vi "Alyssa_GlueLineAndDots.vi"() -> ()   [LabVIEW 2016]
uses:
  C:/Users/Aerotech/Documents/BNLStaveAssembly-blueprint/Bin/Aerotech.A3200.dll
  BNLStaveAssembly-blueprint/Bin/Aerotech.A3200.dll
  <vilib>/vision/Image Controls.llb/IMAQ Image.ctl
  <vilib>/LabVIEW Interface for Arduino/Type Defs/Arduino Resource.ctl
  <vilib>/LabVIEW Interface for Arduino/Type Defs/Board Type.ctl
  <vilib>/LabVIEW Interface for Arduino/Type Defs/Pin Mode.ctl
  <vilib>/Utility/file.llb/Read Delimited Spreadsheet (DBL).vi
  <vilib>/LabVIEW Interface for Arduino/LabVIEW Interface for Arduino.lvlib
panel:
  out "check":dbl[][](array[numeric])
  in  "y dist (mm)":dbl
  in  "How many lines? (actual # will be x2)":i32
  in  "?":T1(tab)
  in  "Module corner coordinates":T2={"X [mm]"=-325.4922095457569, "Y [mm]"=111.42987050829626, "Z [mm] "=34.99996599632762}
  in  "Axis speeds (mm/s)":T3={"vX [mm]"=49.0, "vY [mm]"=49.0, "vZ [mm] "=49.0}
  in  "Home?":bool
  in  "Lowest Z Position":dbl=38.0
  out "Arduino Resource":T4={"VISA resource"="GlueCTRL", "Board Type"=enum."Uno", "Connection Type"=enum."USB / Serial", "Bytes Per Packet (15)"=15}
  in  "Digital I/O Pin":u8=7
  in  "XYZ Stage Control":refnum<k24>
  in  "Testing?":bool
  out "Difference camera/syringe in X":dbl=-133.03368290747076
  out "Difference camera/syringe in y":dbl=-2.170984960815403
  in  "um/pix resolution":dbl=1.58
  in  "Image Feed":T6=refnum
  in  "Path to save collected images":path=path "C:/Users/Aerotech/cernbox/BNL/Stave Assembly Records/2017-06-12/3"
  in  "Estimate distance y":dbl
  in  "Estimate distance x":dbl=130.0
  in  "Lowest Z position Calibration":dbl=17.0
  out "Final Position":T7={"Final X"=-325.49379764644783, "Final Y"=23.533617154160947, "Final Z"=34.99956596392527}
  in  "error in":errorcluster
  out "Arduino Resource 2":T4={"VISA resource"="COM4", "Board Type"=enum."Uno", "Connection Type"=enum."USB / Serial", "Bytes Per Packet (15)"=15}
  out "Module Start":T7
  in  "Digital I/O Pin 2":u8=7
  out "XYZ .NET Refnum out":refnum<k24>
  out "XYZ .NET Refnum out 2":refnum<k24>
  out "error out":errorcluster={"status"=FALSE, "code"=1073676418, "source"="VISA Close in GlueSingleModule(SubVI).vi->2_VisualizeModulePositioning2.vi->VMP_TestStand.vi"}
  # "Overview: This takes a pattern of zeroes/ones (.csv file) as well as the start coordinates of the top left corner of a module and places dots of glue  \nRequirements: NI Arduino dependencies\nInstructions: Select a .csv file (ones indicate regions for glue) as well as a starting coordinate (this is default to the top left corner of the module spacer). You \ncan also input axis speeds (default to maximum) and module lengths and widths (default to 90 mm) which are the widths of the module to which you want to \nplace glue. Lastly, one can choose to Home the stage here and can select the lowest position in Z. The default is that the stage moves down 2-3 mm in Z \nwhile dispensing.  The Arduino inputs are default and simply allow the LabView program to drigger the Arduino (which sends a signal to the dispenser). The \nprogram signals to dispense air- all other parameters such as length of dispensing (default: 350 millisec), pressure (default: 48 psi), and vacuum pressure \n(default: 7.8 psi) are set on the dispenser itself. The defaults are highly recommended here."
  # "Positioning Inputs"
  # "Arduino Inputs"
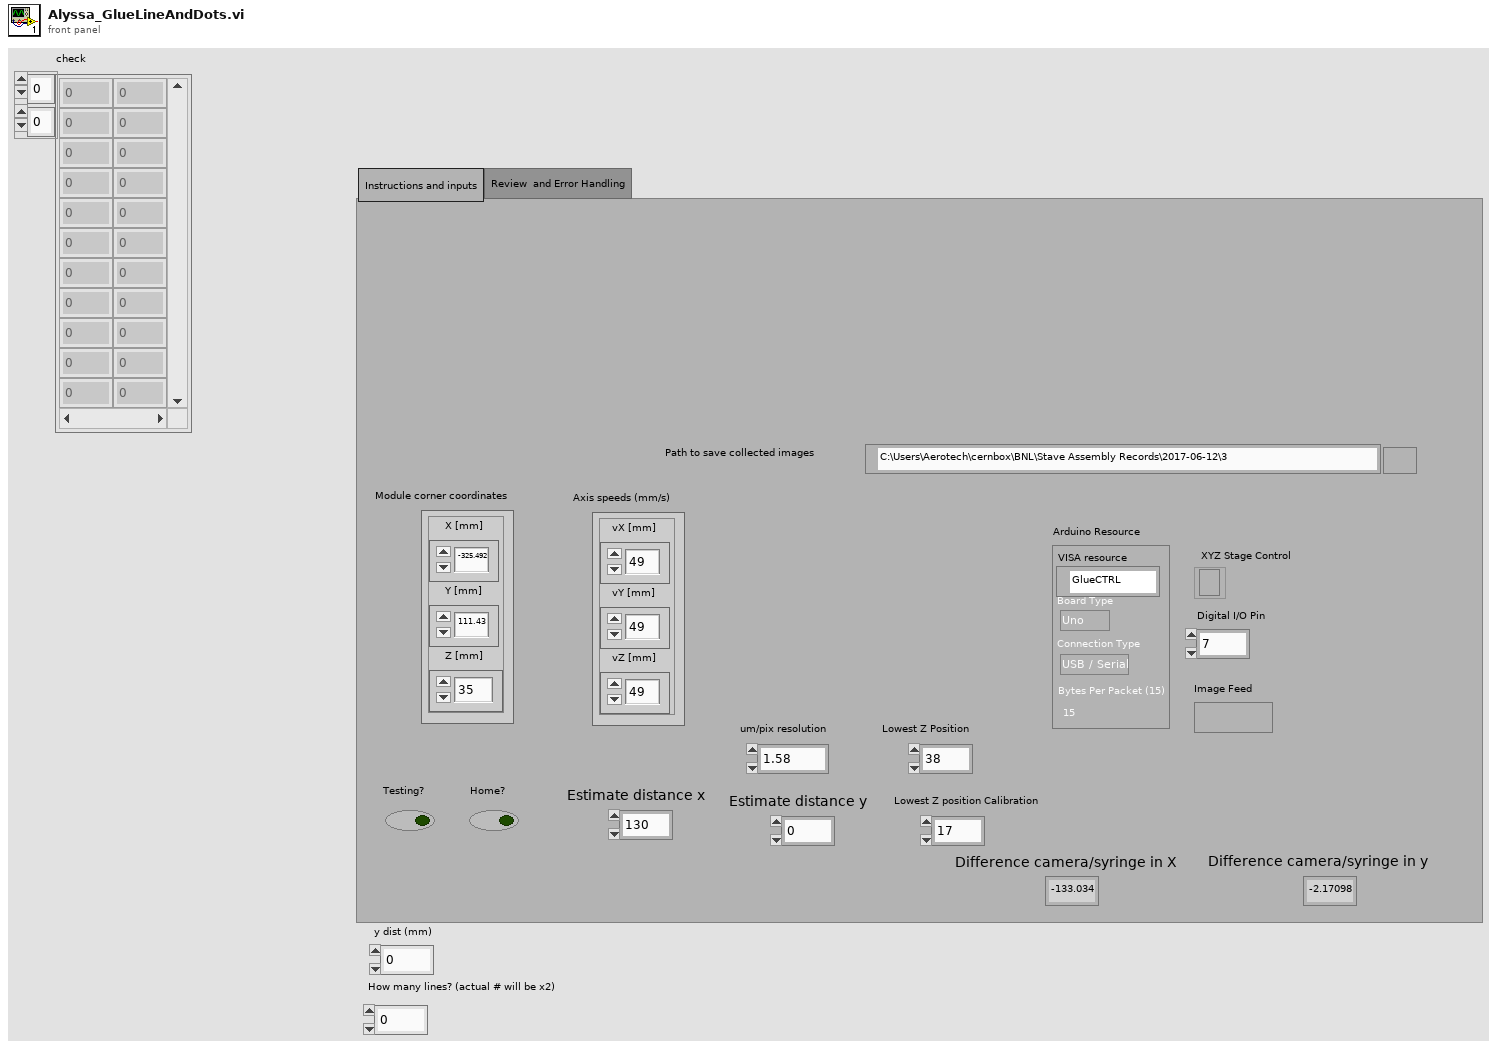
[diagram p1: front panel]
types:
  T1 = enum32{"Instructions and inputs", "Review  and Error Handling"}
  T2 = cluster{"X [mm]":dbl, "Y [mm]":dbl, "Z [mm] ":dbl}
  T3 = cluster{"vX [mm]":dbl, "vY [mm]":dbl, "vZ [mm] ":dbl}
  T4 = typedef "LabVIEW Interface for Arduino.lvlib/Arduino Resource.ctl" = cluster{"VISA resource":refnum<visa-resource-name>, "Board Type":T5, "Connection Type":enum8{"USB / Serial"}, "Bytes Per Packet (15)":u8}
  T5 = typedef "LabVIEW Interface for Arduino.lvlib/Board Type.ctl" = enum16{"Uno", "Dimuelanove w/Atmega 328", "Mega 2560"}
  T6 = typedef "IMAQ Image.ctl" = refnum<image>
  T7 = cluster{"Final X":dbl, "Final Y":dbl, "Final Z":dbl}
  T8 = typedef "LabVIEW Interface for Arduino.lvlib/Pin Mode.ctl" = enum8{"Input", "Output"}
  T9 = cluster{dbl, "Y [mm]":dbl, "Lowest Z Position":dbl}
  T10 = cluster{"Final X":dbl, "Final Y":dbl, "vZ [mm]":dbl}
  T11 = cluster{dbl, "Final Y":dbl, "Lowest Z Position":dbl}
  T12 = cluster{"Final X":dbl, "Final Y":dbl, "Z [mm] ":dbl}
  T13 = cluster{"Final X":dbl, "Final Y":dbl, "Lowest Z Position":dbl}
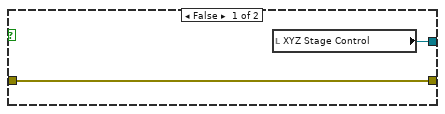
[diagram p3: hidden frame]
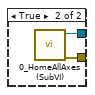
[diagram p4: hidden frame]
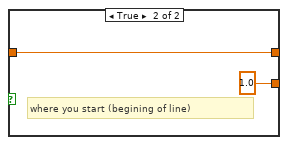
[diagram p6: hidden frame]
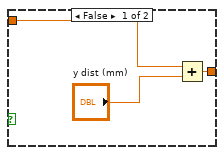
[diagram p7: hidden frame]
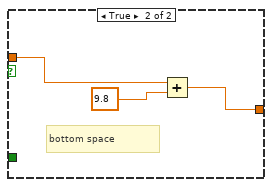
[diagram p8: hidden frame]
diagram:
  n1 = case shown="True" "Testing?" {
    tunnel: [w11 w13] -> w5
    tunnel: [w10 w12] -> w7
    tunnel: "error in" -> [w10 _]
    frame False {
      n2 = local read "XYZ Stage Control"() -> (w11:refnum<k24>)
    }
    frame True {
      n3 = case shown="False" "Home?" {
        tunnel: [w17 w23] -> w13
        tunnel: [w16 w22] -> w12
        frame False {
          w19 = string[] ["X", "Y", "Z"] ("Axes Names")
          n4 = call "Connect.vi"() -> ("error out"=w20:errorcluster, "controller"=w15:refnum<k24>)  [unwired: 10 in]
          n5 = call "EnableMultiple.vi"("error in (no error)"=w20, "axis names"=w19, "controller in"=w15) -> ("error out"=w21:errorcluster, "controller out"=w18:refnum<k24>)  [unwired: 7 in]
          n6 = call "GetCurrentXYZPosition (SubVI).vi"(".NET Refnum in - Device"=w18, "error in (no error)"=w21, "Axes Names"=w19) -> ("error out"=w16:errorcluster, ".NET Refnum out  - Device"=w17:refnum<k24>)  [unwired: 3 in, 4 out]
        }
        frame True {
          n7 = call "0_HomeAllAxes (SubVI).vi"() -> ("error out"=w22:errorcluster, "controller out"=w23:refnum<k24>)  [unwired: 8 in, 2 out]
        }
      }
    }
  }
  n8 = flat-sequence {
    tunnel: [w42] -> w9
    tunnel: w7 -> [w32]
    tunnel: w5 -> [w26]
    tunnel: w9 -> [w203]
    tunnel: [w190] -> w1
    tunnel: [w342] -> w4
    tunnel: [w335] -> w3
    tunnel: [w334] -> w2
    tunnel: w1 -> [w322]
    tunnel: w4 -> [w360]
    tunnel: w3 -> [w346]
    tunnel: w2 -> [w344]
    frame #0 {
      n9 = flat-sequence {
        tunnel: w32 -> [w56]
        tunnel: [w55] -> w27
        tunnel: w26 -> [w49]
        tunnel: w27 -> [w58]
        tunnel: [w57] -> w25
        tunnel: [w77] -> w29
        tunnel: w25 -> [w76]
        tunnel: w29 -> [w137]
        tunnel: [w135] -> w28
        tunnel: [w169] -> w30
        tunnel: w28 -> [w170]
        tunnel: [w168] -> w24
        frame #0 {
          n10 = local read "Module corner coordinates"() -> (w51:T2)
          n11 = Unbundle(w51) -> ("X [mm]"=w48:dbl, "Y [mm]"=w45:dbl)  [unwired: 1 out]
          n12 = local read "Axis speeds (mm/s)"() -> (w54:T3)
          n13 = Add(x=w48, y=133.0) -> (x+y=w46:dbl)
          n14 = Bundle(w46, "Y [mm]"=w45, "Lowest Z Position"="Lowest Z Position") -> (w50:T9)  [unwired: 1 in]
          n15 = Bundle(w46, "Y [mm]"=w45, "Lowest Z Position"="Lowest Z Position") -> (w43:T9)  [unwired: 1 in]
          n16 = call "Go2XYZ (SubVI).vi"(".NET Refnum in"=w49, "Go to Coordinates"=w50, "Axis Speeds"=w54, "error in (no error)"=w56) -> (".NET Refnum out"=w53:refnum<k24>, "Final Position"=→"Final Position":T7, "error out"=w55:errorcluster)  [unwired: 7 in, 2 out]
          n17 = local write "Module corner coordinates"(w43) -> ()
          n18 = local write "XYZ Stage Control"(w53) -> ()
        }
        frame #1 {
          n19 = while {
            tunnel: w58 -> [w75]
            tunnel: [w71] -> w57
            stop <- w74 stop-if-true
            n20 = local read "Module corner coordinates"() -> (w69:T2)
            n21 = call "Lower glue mount"("error in (no error)"=w75) -> ("Move Z down"=w66:dbl, "Move Z up"=w65:dbl, "Accept current Z?"=w74:bool, "error out"=w72:errorcluster)  [unwired: 14 in, 1 out]
            n22 = local read "Lowest Z Position"() -> (w59:dbl)
            n23 = local read "Axis speeds (mm/s)"() -> (w73:T3)
            n24 = local read "XYZ Stage Control"() -> (w61:refnum<k24>)
            n25 = Add(x=w59, y=w66) -> (x+y=w63:dbl)
            n26 = Subtract(x=w63, y=w65) -> (x-y=w62:dbl)
            n27 = Unbundle(w69) -> ("X [mm]"=w68:dbl, "Y [mm]"=w67:dbl)  [unwired: 1 out]
            n28 = Bundle("X [mm]"=w68, "Y [mm]"=w67, w62) -> (w64:cluster{"X [mm]":dbl, "Y [mm]":dbl, dbl})  [unwired: 1 in]
            n29 = local write "Lowest Z Position"(w62) -> ()
            n30 = call "Go2XYZ (SubVI).vi"(".NET Refnum in"=w61, "Go to Coordinates"=w64, "Axis Speeds"=w73, "error in (no error)"=w72) -> (".NET Refnum out"=w70:refnum<k24>, "Final Position"=w60:T7, "error out"=w71:errorcluster)  [unwired: 7 in, 2 out]
            n31 = local write "XYZ Stage Control"(w70) -> ()
            n32 = local write "Final Position"(w60) -> ()
          }
        }
        frame #2 {
          n33 = call "Calibrate distance?"("error in (no error)"=w76) -> ("Calibrate distance?"=w78:bool, "error out"=w79:errorcluster)  [unwired: 16 in, 1 out]
          n34 = case shown="True" w78 {
            tunnel: w79 -> [w80 w82]
            tunnel: [w80 w83] -> w77
            frame False {
            }
            frame True {
              n35 = flat-sequence {
                tunnel: w82 -> [w85]
                tunnel: [w84] -> w81
                frame #0 {
                  n36 = local read "Final Position"() -> (w92:T7)
                  n37 = local read "Axis speeds (mm/s)"() -> (w88:T3)
                  n38 = local read "XYZ Stage Control"() -> (w87:refnum<k24>)
                  n39 = Unbundle(w92) -> ("Final X"=w90:dbl, "Final Y"=w91:dbl)  [unwired: 1 out]
                  n40 = Bundle("Final X"=w90, "Final Y"=w91, "vZ [mm]"=-20.0) -> (w94:T10)  [unwired: 1 in]
                  n41 = call "Go2XYZ (SubVI).vi"(".NET Refnum in"=w87, "Go to Coordinates"=w94, "Axis Speeds"=w88, "error in (no error)"=w85) -> (".NET Refnum out"=w86:refnum<k24>, "Final Position"=w89:T7, "error out"=w84:errorcluster)  [unwired: 7 in, 2 out]
                  n42 = local write "XYZ Stage Control"(w86) -> ()
                  n43 = local write "Final Position"(w89) -> ()
                }
              }
              n44 = while {
                tunnel: [w133] -> w83
                tunnel: w81 -> [w121]
                i -> [w118]
                stop <- w134 stop-if-true
                n45 = local read "Final Position"() -> (w95:T7)
                n46 = Unbundle(w95) -> ("Final X"=w100:dbl, "Final Y"=w98:dbl, "Final Z"=w99:dbl)
                n47 = local read "Testing?"() -> (w116:bool)
                n48 = local read "Axis speeds (mm/s)"() -> (w123:T3)
                n49 = local read "XYZ Stage Control"() -> (w119:refnum<k24>)
                n50 = Subtract(x=w98, y=220.0) -> (x-y=w96:dbl)
                n51 = Equal To 0?(x=w118) -> (x = 0?=w117:bool)
                n52 = And(x=w116, y=w117) -> (x .and. y?=w115:bool)
                n53 = Bundle("Final X"=w100, w96, "Final Z"=w99) -> (w101:cluster{"Final X":dbl, dbl, "Final Z":dbl})  [unwired: 1 in]
                n54 = call "CalibrateDistanceCameraSyringe.vi"("Path to save collected images"="Path to save collected images", "Image Feed"="Image Feed", "Off stave position"=w101, ".NET Refnum in"=w119, "Axis speeds (mm/s)"=w123, "Lowest Z Position"="Lowest Z position Calibration", "Estimate distance y"="Estimate distance y", "um/pix resolution"="um/pix resolution", "Estimate distance x"="Estimate distance x", "error in"=w121, "Testing?"=w115) -> ("XYZ .NET Refnum out"=w122:refnum<k24>, "error out"=w120:errorcluster, "X/Y difference (CAMERA - SYRINGE)"=w130:dbl[][])  [unwired: 2 in]
                n55 = local read "Difference camera/syringe in X"() -> (w105:dbl)
                n56 = local read "Difference camera/syringe in y"() -> (w102:dbl)
                n57 = local read "Lowest Z position Calibration"() -> (w107:dbl)
                n58 = call "Accept calibration?"("error in (no error)"=w120) -> ("Change in lowest Z"=w109:dbl, "Change in distance Y estimate"=w110:dbl, "Change in distance X estimate"=w111:dbl, "Accept the distance syringe/camera?"=w134:bool, "error out"=w133:errorcluster)  [unwired: 13 in, 1 out]
                n59 = local write "XYZ Stage Control"(w122) -> ()
                n60 = Index Array(array=w130, index (row) #1=0 ("index (row)"), index (col) #1=0 ("disabled index (col)"), index (row) #2=0 ("index (row)"), index (col) #2=1 ("disabled index (col)")) -> (element #1=→"Difference camera/syringe in X":dbl, element #2=→"Difference camera/syringe in y":dbl)
                n61 = Add(x=w105, y=w111) -> (x+y=w104:dbl)
                n62 = Add(x=w102, y=w110) -> (x+y=w103:dbl)
                n63 = Add(x=w107, y=w109) -> (x+y=w108:dbl)
                n64 = local write "Difference camera/syringe in X"(w104) -> ()
                n65 = local write "Difference camera/syringe in y"(w103) -> ()
                n66 = local write "Lowest Z position Calibration"(w108) -> ()
              }
            }
          }
        }
        frame #3 {
          n67 = flat-sequence {
            tunnel: w137 -> [w144]
            tunnel: [w141] -> w136
            tunnel: [w155] -> w135
            tunnel: w136 -> [w156]
            frame #0 {
              n68 = local read "Module corner coordinates"() -> (w154:T2)
              n69 = local read "Difference camera/syringe in y"() -> (w149:dbl)
              n70 = local read "Difference camera/syringe in X"() -> (w150:dbl)
              n71 = Unbundle By Name(w154) -> ("X [mm]"=w140:dbl, "Y [mm]"=w153:dbl)  [unwired: 1 out]
              n72 = Subtract(x=w153, y=w149) -> (x-y=w151:dbl)
              n73 = Subtract(x=w140, y=133.0) -> (x-y=w138:dbl)
              n74 = local read "Axis speeds (mm/s)"() -> (w145:T3)
              n75 = local read "XYZ Stage Control"() -> (w146:refnum<k24>)
              n76 = Subtract(x=w138, y=w150) -> (x-y=w152:dbl)
              n77 = Bundle(w152, w151, "index (row)"=-20.0) -> (w143:cluster{dbl, dbl, "index (row)":dbl})  [unwired: 1 in]
              n78 = call "Go2XYZ (SubVI).vi"(".NET Refnum in"=w146, "Go to Coordinates"=w143, "Axis Speeds"=w145, "error in (no error)"=w144) -> (".NET Refnum out"=w147:refnum<k24>, "Final Position"=w148:T7, "error out"=w141:errorcluster)  [unwired: 7 in, 2 out]
              n79 = local write "XYZ Stage Control"(w147) -> ()
              n80 = local write "Module corner coordinates"(w148) -> ()
            }
            frame #1 {
              n81 = local read "Module corner coordinates"() -> (w161:T2)
              n82 = local read "Lowest Z Position"() -> (w164:dbl)
              n83 = local read "Axis speeds (mm/s)"() -> (w158:T3)
              n84 = local read "XYZ Stage Control"() -> (w157:refnum<k24>)
              n85 = Unbundle(w161) -> ("X [mm]"=w162:dbl, "Y [mm]"=w163:dbl)  [unwired: 1 out]
              n86 = Subtract(x=w164, y=2.0) -> (x-y=w166:dbl)
              n87 = Bundle("X [mm]"=w162, "Y [mm]"=w163, w166) -> (w167:cluster{"X [mm]":dbl, "Y [mm]":dbl, dbl})  [unwired: 1 in]
              n88 = call "Go2XYZ (SubVI).vi"(".NET Refnum in"=w157, "Go to Coordinates"=w167, "Axis Speeds"=w158, "error in (no error)"=w156) -> (".NET Refnum out"=w159:refnum<k24>, "Final Position"=w160:T7, "error out"=w155:errorcluster)  [unwired: 7 in, 2 out]
              n89 = local write "XYZ Stage Control"(w159) -> ()
              n90 = local write "Module corner coordinates"(w160) -> ()
            }
          }
        }
        frame #4 {
          n91 = while {
            tunnel: w170 -> [w184]
            tunnel: [w186] -> w169
            tunnel: [w171] -> w168
            stop <- w172 continue-if-true
            n92 = local read "Module corner coordinates"() -> (w183:T2)
            n93 = call "Ready to glue?"("error in (no error)"=w184) -> ("Move in Z"=w180:dbl, "Move in Y"=w181:dbl, "Move in X"=w182:dbl, "Oh yeah! Reset Arduino and go!"=w172:bool, "error out"=w185:errorcluster)  [unwired: 13 in, 1 out]
            n94 = local read "Axis speeds (mm/s)"() -> (w189:T3)
            n95 = local read "XYZ Stage Control"() -> (w187:refnum<k24>)
            n96 = Unbundle(w183) -> ("X [mm]"=w179:dbl, "Y [mm]"=w178:dbl, "Z [mm]"=w177:dbl)
            n97 = Add(x=w179, y=w182) -> (x+y=w174:dbl)
            n98 = Add(x=w178, y=w181) -> (x+y=w176:dbl)
            n99 = Add(x=w177, y=w180) -> (x+y=w175:dbl)
            n100 = Bundle(w174, w176, w175) -> (w173:cluster{dbl, dbl, dbl})  [unwired: 1 in]
            n101 = call "Go2XYZ (SubVI).vi"(".NET Refnum in"=w187, "Go to Coordinates"=w173, "Axis Speeds"=w189, "error in (no error)"=w185) -> (".NET Refnum out"=w188:refnum<k24>, "Final Position"=w171:T7, "error out"=w186:errorcluster)  [unwired: 7 in, 2 out]
            n102 = local write "XYZ Stage Control"(w188) -> ()
            n103 = local write "Final Position"(w171) -> ()
            n104 = local write "Module corner coordinates"(w171) -> ()
          }
        }
      }
      n105 = local read "Digital I/O Pin"() -> (w31:u8)
      n106 = call <vilib>:"Init.vi"("VISA resource"=refnum<visa-resource-name> "GlueCTRL", "error in"=w30) -> ("Arduino Resource"=w34:T4, "error out"=w35:errorcluster)  [unwired: 16 in]
      "Arduino Resource" <- w34
      n107 = call <vilib>:"Set Digital Pin Mode.vi"("Arduino Resource"=w34, "Digital I/O Pin"="Digital I/O Pin", "Pin Mode (Input)"=Pin_Mode."Output", "error in"=w35) -> ("Arduino Resource"=w38:T4, "error out"=w39:errorcluster)  [unwired: 10 in]
      n108 = call <vilib>:"Digital Write Pin.vi"("Arduino Resource"=w38, "Digital I/O Pin (0)"=w31, "Value (0)"=u8 0, "error in"=w39) -> ("Arduino Resource"=w33:T4, "error out"=w42:errorcluster)  [unwired: 10 in]
      n109 = local write "Arduino Resource"(w33) -> ()
      "Module Start" <- w24
    }
    frame #1 {
      n110 = local read "Module corner coordinates"() -> (w202:T2)
      n111 = Unbundle By Name(w202) -> ("X [mm]"=w200:dbl, "Y [mm]"=w199:dbl, "Z [mm]"=w198:dbl)
      n112 = for {
        N: "How many lines? (actual # will be x2)" -> [_]
        tunnel: w203 -> [w217]
        tunnel: [w216] -> w191
        shift-right: [w214] -> _
        shift-left: w199 -> [w215]
        tunnel: w198 -> [w213]
        shift-right: [w212] -> _
        shift-left: w200 -> [w211]
        i -> [w206]
        n113 = local read "How many lines? (actual # will be x2)"() -> (w209:i32)
        n114 = Subtract(x=w209, y=2) -> (x-y=w207:i32)
        n115 = Equal?(x=w206, y=w207) -> (x = y?=w204:bool)
        n116 = Equal To 0?(x=w206) -> (x = 0?=w205:bool)
        n117 = for {
          N: 2 -> [_]
          tunnel: w217 -> [w239]
          tunnel: [w237] -> w216
          shift-right: [w236] -> w214
          shift-left: w215 -> [w226]
          tunnel: w205 -> [w227]
          tunnel: w213 -> [w225]
          tunnel: w211 -> [w228]
          tunnel: [w223] -> w212
          tunnel: w204 -> [w218]
          i -> [w224]
          # "move to starting y position"
          # "go back up in z and stop gluing"
          # "move down in z and over in x while gluing"
          n118 = flat-sequence {
            tunnel: w239 -> [w257]
            tunnel: [w243] -> w234
            tunnel: [w257] -> w233
            tunnel: [w249] -> w232
            tunnel: [w248] -> w231
            tunnel: [w251] -> w230
            tunnel: [w249] -> w229
            tunnel: w228 -> [w247]
            tunnel: w227 -> [w242]
            tunnel: w226 -> [w252]
            tunnel: w225 -> [w251]
            tunnel: w224 -> [w250]
            tunnel: w218 -> [w246]
            tunnel: [w286] -> w221
            tunnel: [w276] -> w220
            tunnel: [w287] -> w219
            tunnel: w229 -> [w287]
            tunnel: w230 -> [w284]
            tunnel: w231 -> [w285]
            tunnel: w232 -> [w277]
            tunnel: w233 -> [w280]
            tunnel: w234 -> [w286]
            tunnel: [w301] -> w241
            tunnel: [w300] -> w240
            tunnel: [w299] -> w238
            tunnel: [w291] -> w235
            tunnel: w221 -> [w289]
            tunnel: w220 -> [w288]
            tunnel: w219 -> [w291]
            tunnel: [w289] -> w222
            tunnel: [w321] -> w237
            tunnel: w238 -> [w307]
            tunnel: w240 -> [w320]
            tunnel: w241 -> [w318]
            tunnel: [w306] -> w236
            tunnel: w235 -> [w306]
            tunnel: [w305] -> w223
            tunnel: w222 -> [w305]
            frame #0 {
              # "where you move in x"
              n119 = Equal To 0?(x=w250) -> (x = 0?=w244:bool)
              n120 = And(x=w244, y=w246) -> (x .and. y?=w245:bool)
              n121 = And(x=w244, y=w242) -> (x .and. y?=w256:bool)
              n122 = case shown="False" w244 {
                tunnel: [0.0 1.0] -> w255
                tunnel: [w259 w262] -> w248
                tunnel: w247 -> [w260 w262]
                frame False {
                  # "where you start (end of line)"
                  n123 = Add(x=w260, y=90 ("x")) -> (x+y=w259:dbl)
                }
                frame True {
                  # "where you start (begining of line)"
                }
              }
              n124 = case shown="False" w256 {
                tunnel: w252 -> [w266 w275]
                tunnel: [w265 w274] -> w249
                tunnel: w245 -> [w264 _]
                frame False {
                  n125 = case shown="True" w264 {
                    tunnel: w266 -> [w269 w272]
                    tunnel: [w268 w270] -> w265
                    frame False {
                      n126 = Add(x=w269, y="y dist (mm)") -> (x+y=w268:dbl)
                    }
                    frame True {
                      # "middle space"
                      n127 = Add(x=w272, y=13.0) -> (x+y=w270:dbl)
                    }
                  }
                }
                frame True {
                  # "bottom space"
                  n128 = Add(x=w275, y=9.8) -> (x+y=w274:dbl)
                }
              }
              n129 = Multiply(x=90, y=w255) -> (x*y=w254:dbl)
              n130 = Add(x=w247, y=w254) -> (x+y=w243:dbl)
            }
            frame #1 {
              n131 = local read "Axis speeds (mm/s)"() -> (w282:T3)
              n132 = local read "XYZ Stage Control"() -> (w279:refnum<k24>)
              n133 = Bundle("X [mm]"=w285, w277, "Z [mm]"=w284) -> (w283:cluster{"X [mm]":dbl, dbl, "Z [mm] ":dbl})  [unwired: 1 in]
              n134 = call "Go2XYZ (SubVI).vi"(".NET Refnum in"=w279, "Go to Coordinates"=w283, "Axis Speeds"=w282, "error in (no error)"=w280) -> (".NET Refnum out"=w278:refnum<k24>, "Final Position"=w281:T7, "error out"=w276:errorcluster)  [unwired: 7 in, 2 out]
              n135 = local write "XYZ Stage Control"(w278) -> ()
              n136 = local write "Final Position"(w281) -> ()
            }
            frame #2 {
              n137 = local read "Final Position"() -> (w292:T7)
              n138 = local read "Arduino Resource"() -> (w302:T4)
              n139 = local read "XYZ Stage Control"() -> (w296:refnum<k24>)
              n140 = local read "Lowest Z Position"() -> (w298:dbl)
              n141 = local read "Digital I/O Pin"() -> (w301:u8)
              n142 = local read "Axis speeds (mm/s)"() -> (w295:T3)
              n143 = Unbundle(w292) -> ("Final Y"=w290:dbl)  [unwired: 2 out]
              n144 = Bundle(w289, "Final Y"=w290, "Lowest Z Position"=w298) -> (w294:T11)  [unwired: 1 in]
              n145 = call <vilib>:"Digital Write Pin.vi"("Arduino Resource"=w302, "Digital I/O Pin (0)"=w301, "Value (0)"=u8 1, "error in"=w288) -> ("Arduino Resource"=w300:T4, "error out"=w299:errorcluster)  [unwired: 10 in]
              n146 = call "Go2XYZ (SubVI).vi"(".NET Refnum in"=w296, "Go to Coordinates"=w294, "Axis Speeds"=w295) -> (".NET Refnum out"=w297:refnum<k24>, "Final Position"=w293:T7)  [unwired: 8 in, 3 out]
              n147 = local write "XYZ Stage Control"(w297) -> ()
              n148 = local write "Arduino Resource"(w300) -> ()
              n149 = local write "Final Position"(w293) -> ()
            }
            frame #3 {
              n150 = local read "Module corner coordinates"() -> (w315:T2)
              n151 = call <vilib>:"Digital Write Pin.vi"("Arduino Resource"=w320, "Digital I/O Pin (0)"=w318, "Value (0)"=u8 0, "error in"=w307) -> ("Arduino Resource"=w317:T4, "error out"=w321:errorcluster)  [unwired: 10 in]
              n152 = local write "Arduino Resource"(w317) -> ()
              n153 = local read "Final Position"() -> (w316:T7)
              n154 = local read "Axis speeds (mm/s)"() -> (w310:T3)
              n155 = local read "XYZ Stage Control"() -> (w309:refnum<k24>)
              n156 = Unbundle(w316) -> ("Final X"=w314:dbl, "Final Y"=w313:dbl)  [unwired: 1 out]
              n157 = Unbundle(w315) -> ("Z [mm]"=w312:dbl)  [unwired: 2 out]
              n158 = Bundle("Final X"=w314, "Final Y"=w313, "Z [mm]"=w312) -> (w311:T12)  [unwired: 1 in]
              n159 = call "Go2XYZ (SubVI).vi"(".NET Refnum in"=w309, "Go to Coordinates"=w311, "Axis Speeds"=w310) -> (".NET Refnum out"=→"XYZ .NET Refnum out":refnum<k24>, "Final Position"=w308:T7)  [unwired: 8 in, 3 out]
              n160 = local write "Final Position"(w308) -> ()
            }
          }
        }
      }
      n161 = local read "Arduino Resource"() -> (w193:T4)
      n162 = local read "Digital I/O Pin"() -> (w192:u8)
      n163 = call <vilib>:"Digital Write Pin.vi"("Arduino Resource"=w193, "Digital I/O Pin (0)"=w192, "error in"=w191) -> ("Arduino Resource"=w196:T4, "error out"=w195:errorcluster)  [unwired: 11 in]
      n164 = call <vilib>:"Close.vi"("Arduino Resource"=w196, "error in"=w195) -> ("error out"=w194:errorcluster)  [unwired: 13 in]
      n165 = VISA Close(VISA resource name=refnum<visa-resource-name> "GlueCTRL", error in (no error)=w194) -> (error out=w190:errorcluster)
    }
    frame #2 {
      n166 = local read "Digital I/O Pin 2"() -> (w324:u8)
      n167 = call <vilib>:"Init.vi"("VISA resource"=refnum<visa-resource-name> "COM4", "error in"=w322) -> ("Arduino Resource"=w326:T4, "error out"=w327:errorcluster)  [unwired: 16 in]
      "Arduino Resource 2" <- w326
      n168 = call <vilib>:"Set Digital Pin Mode.vi"("Arduino Resource"=w326, "Digital I/O Pin"="Digital I/O Pin 2", "Pin Mode (Input)"=Pin_Mode."Output", "error in"=w327) -> ("Arduino Resource"=w330:T4, "error out"=w331:errorcluster)  [unwired: 10 in]
      n169 = call <vilib>:"Digital Write Pin.vi"("Arduino Resource"=w330, "Digital I/O Pin (0)"=w324, "Value (0)"=u8 0, "error in"=w331) -> ("Arduino Resource"=w325:T4, "error out"=w323:errorcluster)  [unwired: 10 in]
      n170 = local write "Arduino Resource 2"(w325) -> ()
      n171 = call "Phase Two!"("error in (no error)"=w323) -> ("error out"=w342:errorcluster)  [unwired: 17 in, 1 out]
      n172 = call-poly <vilib>:"Read Delimited Spreadsheet.vi"("file path (dialog if empty)"=path "C:/Users/Aerotech/Documents/alyssa/DotTest.csv", "number of rows (all:-1)"=-1, "delimiter (\\t)"="," ("delimiter (\\t)")) -> ("all rows"=w337:dbl[][])  [unwired: 7 in, 5 out]
      "check" <- w337
      n173 = Index Array(array=w337, index (col) #1=0 ("index"), index (col) #2=1 ("index")) -> (element #1=w335:dbl[], element #2=w334:dbl[])  [unwired: 2 in]
    }
    frame #3 {
      n174 = local read "Module corner coordinates"() -> (w361:T2)
      n175 = Reverse 1D Array(array=w346) -> (reversed array=w345:dbl[])
      n176 = Reverse 1D Array(array=w344) -> (reversed array=w343:dbl[])
      n177 = Unbundle By Name(w361) -> ("X [mm]"=w359:dbl, "Y [mm]"=w358:dbl, "Z [mm]"=w355:dbl)
      n178 = Add(x=w343, y=w358) -> (x+y=w356:dbl[])
      n179 = Add(x=w345, y=w359) -> (x+y=w357:dbl[])
      n180 = for {
        tunnel: w360 -> [w374]
        tunnel: [w373] -> w347
        tunnel: w357 -> [w368] mode=indexing
        tunnel: w356 -> [w367] mode=indexing
        tunnel: w355 -> [w366]
        n181 = flat-sequence {
          tunnel: [w378] -> w372
          tunnel: w374 -> [w378]
          tunnel: w368 -> [w380]
          tunnel: w367 -> [w379]
          tunnel: w366 -> [w376]
          tunnel: [w377] -> w365
          tunnel: [w376] -> w362
          tunnel: [w397] -> w369
          tunnel: [w396] -> w370
          tunnel: [w388] -> w371
          tunnel: w372 -> [w390]
          tunnel: w365 -> [w387]
          tunnel: [w386] -> w364
          tunnel: [w385] -> w363
          tunnel: w362 -> [w385]
          tunnel: [w414] -> w373
          tunnel: w371 -> [w404]
          tunnel: w370 -> [w413]
          tunnel: w369 -> [w411]
          tunnel: w364 -> [w401]
          tunnel: w363 -> [w400]
          frame #0 {
            n182 = local read "Axis speeds (mm/s)"() -> (w383:T3)
            n183 = local read "XYZ Stage Control"() -> (w382:refnum<k24>)
            n184 = Bundle(w380, w379, "Z [mm]"=w376) -> (w375:cluster{dbl, dbl, "Z [mm] ":dbl})  [unwired: 1 in]
            n185 = call "Go2XYZ (SubVI).vi"(".NET Refnum in"=w382, "Go to Coordinates"=w375, "Axis Speeds"=w383) -> (".NET Refnum out"=w381:refnum<k24>, "Final Position"=w377:T7)  [unwired: 8 in, 3 out]
            n186 = local write "XYZ Stage Control"(w381) -> ()
            n187 = local write "Final Position"(w377) -> ()
          }
          frame #1 {
            n188 = local read "Arduino Resource 2"() -> (w398:T4)
            n189 = local read "Lowest Z Position"() -> (w395:dbl)
            n190 = local read "Digital I/O Pin 2"() -> (w397:u8)
            n191 = local read "Axis speeds (mm/s)"() -> (w392:T3)
            n192 = local read "XYZ Stage Control"() -> (w393:refnum<k24>)
            n193 = Unbundle(w387) -> ("Final X"=w389:dbl, "Final Y"=w391:dbl)  [unwired: 1 out]
            n194 = Bundle("Final X"=w389, "Final Y"=w391, "Lowest Z Position"=w395) -> (w384:T13)  [unwired: 1 in]
            n195 = call <vilib>:"Digital Write Pin.vi"("Arduino Resource"=w398, "Digital I/O Pin (0)"=w397, "Value (0)"=u8 1, "error in"=w390) -> ("Arduino Resource"=w396:T4, "error out"=w388:errorcluster)  [unwired: 10 in]
            n196 = call "Go2XYZ (SubVI).vi"(".NET Refnum in"=w393, "Go to Coordinates"=w384, "Axis Speeds"=w392) -> (".NET Refnum out"=w394:refnum<k24>, "Final Position"=w386:T7)  [unwired: 8 in, 3 out]
            n197 = local write "XYZ Stage Control"(w394) -> ()
            n198 = local write "Arduino Resource 2"(w396) -> ()
          }
          frame #2 {
            n199 = call <vilib>:"Digital Write Pin.vi"("Arduino Resource"=w413, "Digital I/O Pin (0)"=w411, "Value (0)"=u8 0, "error in"=w404) -> ("Arduino Resource"=w403:T4, "error out"=w414:errorcluster)  [unwired: 10 in]
            n200 = local write "Arduino Resource 2"(w403) -> ()
            n201 = local read "Axis speeds (mm/s)"() -> (w407:T3)
            n202 = local read "XYZ Stage Control"() -> (w406:refnum<k24>)
            n203 = Unbundle(w401) -> ("Final X"=w410:dbl, "Final Y"=w409:dbl)  [unwired: 1 out]
            n204 = Bundle("Final X"=w410, "Final Y"=w409, "Z [mm]"=w400) -> (w408:T12)  [unwired: 1 in]
            n205 = call "Go2XYZ (SubVI).vi"(".NET Refnum in"=w406, "Go to Coordinates"=w408, "Axis Speeds"=w407) -> (".NET Refnum out"=→"XYZ .NET Refnum out 2":refnum<k24>, "Final Position"=w405:T7)  [unwired: 8 in, 3 out]
            n206 = local write "Final Position"(w405) -> ()
          }
        }
      }
      n207 = local read "Arduino Resource 2"() -> (w349:T4)
      n208 = local read "Digital I/O Pin 2"() -> (w348:u8)
      n209 = call <vilib>:"Digital Write Pin.vi"("Arduino Resource"=w349, "Digital I/O Pin (0)"=w348, "error in"=w347) -> ("Arduino Resource"=w353:T4, "error out"=w352:errorcluster)  [unwired: 11 in]
      n210 = call <vilib>:"Close.vi"("Arduino Resource"=w353, "error in"=w352) -> ("error out"=w351:errorcluster)  [unwired: 13 in]
      n211 = VISA Close(VISA resource name=refnum<visa-resource-name> "GlueCTRL", error in (no error)=w351) -> (error out=→"error out":errorcluster)
    }
  }
  n212 = disable-structure shown="Disabled" {
    frame Disabled {
      n213 = local read "XYZ Stage Control"() -> (w422:refnum<k24>)
      n214 = local read "Final Position"() -> (w418:T7)
      n215 = local read "Lowest Z Position"() -> (w416:dbl)
      n216 = Bundle("Lowest Z Position"=w416) -> (w415:cluster{void, void, "Lowest Z Position":dbl}, w417)  [unwired: 2 in]
      n217 = local read "Axis speeds (mm/s)"() -> (w419:T3)
      n218 = call "Go2XYZ (SubVI).vi"(".NET Refnum in"=w422, "Go to Coordinates"=w415, "Axis Speeds"=w419) -> (".NET Refnum out"=w421:refnum<k24>, "Final Position"=w420:T7)  [unwired: 8 in, 3 out]
      n219 = local write "XYZ Stage Control"(w421) -> ()
      n220 = local write "Final Position"(w420) -> ()
    }
    frame Enabled {
    }
  }
